vi "UHR-Fleezers Control (host) - 12.2.vi"() -> ()   [LabVIEW 2014] (continued)
          frame #3 {
            n2188 = Wait (ms)(milliseconds to wait=u32 500) -> ()  [unwired: 1 out]
          }
          frame #4 {
            n2189 = property on="Trap Pos. FB ON" class="Bool (strict)"("Val(Sgnl)"=TRUE ("Value (Signaling)")) -> ()  [unwired: 2 in, 2 out]
            n2190 = Wait (ms)(milliseconds to wait=u32 250) -> ()  [unwired: 1 out]
          }
          frame #5 {
            n2191 = case shown="\"1\"" "Remove Action Offset Dropdown" {
              tunnel: TRUE ("Value (Signaling)") -> [w3127 w3135 w3143]
              frame "1" {
                n2192 = flat-sequence {
                  tunnel: w3127 -> [w3134]
                  frame #0 {
                    n2193 = local read "factor"() -> (w3129:dbl)
                    n2194 = Greater Than 0?(x=w3129) -> (x > 0?=w3133:bool)
                    n2195 = Select(t=1.0, s=w3133, f=-1.0) -> (s? t:f=w3130:dbl)
                    n2196 = Multiply(x=w3130, y=w3129) -> (x*y=w3128:dbl)
                    n2197 = local write "factor"(w3128) -> ()
                  }
                  frame #1 {
                    n2198 = property on="Remove Offset to factor" class="Bool (strict)"("Val(Sgnl)"=w3134) -> ()  [unwired: 2 in, 2 out]
                  }
                }
              }
              frame "2" {
                n2199 = flat-sequence {
                  tunnel: w3135 -> [w3142]
                  frame #0 {
                    n2200 = local read "factor"() -> (w3136:dbl)
                    n2201 = Greater Than 0?(x=w3136) -> (x > 0?=w3141:bool)
                    n2202 = Select(t=-1.0, s=w3141, f=1.0) -> (s? t:f=w3139:dbl)
                    n2203 = Multiply(x=w3136, y=w3139) -> (x*y=w3138:dbl)
                    n2204 = local write "factor"(w3138) -> ()
                  }
                  frame #1 {
                    n2205 = property on="Remove Offset to factor" class="Bool (strict)"("Val(Sgnl)"=w3142) -> ()  [unwired: 2 in, 2 out]
                  }
                }
              }
              frame "0", Default {
                n2206 = property on="Remove Action Offset" class="Bool (strict)"("Val(Sgnl)"=w3143) -> ()  [unwired: 2 in, 2 out]
              }
            }
            n2207 = case shown="False" "Trap Trig Fl." {
              frame False {
                n2208 = case shown="True" "Green ON after FB ON?" {
                  selector: "Green ON after FB ON?" -> [_ w3145]
                  frame False {
                  }
                  frame True {
                    n2209 = property on="Green ON/Interlacing" class="Bool (strict)"("Val(Sgnl)"=w3145) -> ()  [unwired: 2 in, 2 out]
                  }
                }
              }
              frame True {
              }
            }
            n2210 = Wait (ms)(milliseconds to wait=u32 250) -> ()  [unwired: 1 out]
          }
          frame #6 {
            n2211 = property on="Start Saving" class="Bool (strict)"("Val(Sgnl)"=TRUE ("Value (Signaling)")) -> ()  [unwired: 2 in, 2 out]
            n2212 = Wait (ms)(milliseconds to wait=u32 5000) -> ()  [unwired: 1 out]
          }
          frame #7 {
            w3149 = TRUE ("Value (Signaling)")
            n2213 = property on="Rem fb disp offset" class="Bool (strict)"("Val(Sgnl)"=w3149) -> ()  [unwired: 2 in, 2 out]
            n2214 = property on="Remove Offset" class="Bool (strict)"("Val(Sgnl)"=w3149) -> ()  [unwired: 2 in, 2 out]
            n2215 = Wait (ms)(milliseconds to wait=u32 100) -> ()  [unwired: 1 out]
          }
          frame #8 {
            n2216 = case shown="True" w3152 {
              frame False {
              }
              frame True {
                n2217 = local write "Trap Trig. Fl."(TRUE ("Value (Signaling)")) -> ()
              }
            }
          }
          frame #9 {
            n2218 = local read "Tether"() -> (w3155:bool)
            n2219 = And(x="Start dipping after?", y=w3155) -> (x .and. y?=w3154:bool)
            n2220 = case shown="True" w3154 {
              frame False {
              }
              frame True {
                n2221 = flat-sequence {
                  frame #0 {
                    n2222 = Multiply(x="Delay before dipping (s)", y=1000.0) -> (x*y=w3158:dbl)
                    n2223 = Wait (ms)(milliseconds to wait=w3158) -> ()  [unwired: 1 out]
                  }
                  frame #1 {
                    n2224 = property on="Dip for Protein" class="Bool (strict)"("Val(Sgnl)"=TRUE ("Value (Signaling)")) -> ()  [unwired: 2 in, 2 out]
                    n2225 = local write "Scripts"(T35."Dipping") -> ()
                  }
                }
              }
            }
          }
        }
      }
      event "Rupture Script": Value Change {
        n2226 = event-data() -> ()  [unwired: 1 in, 5 out]
        n2227 = local write "Rupture Script"(FALSE ("Rupture Script")) -> ()
        n2228 = flat-sequence {
          frame #0 {
            w3164 = TRUE
            w3169 = FALSE
            # "Number 6 for now is the\nrupture-experiment\nparameters."
            n2229 = local read "Starting Trap D (MHz)"() -> (w3170:dbl)
            n2230 = local write "Restart DMA? (AOD)"(w3169) -> ()
            n2231 = Replace Array Subset(array=u32[] [0] ("Index Values"), new element=6, index=0) -> (w3165:u32[])
            n2232 = local write "Save scans"(w3169) -> ()
            n2233 = property on="Trap D (MHz)" class="DigNum (strict)"("Val(Sgnl)"=w3170) -> ()  [unwired: 2 in, 2 out]
            n2234 = property on="Saved AOD Raster Scan Parameter Sets" class="Arr (strict)"("Index Values"=w3165) -> ()  [unwired: 2 in, 2 out]
            n2235 = property on="Start Saving" class="Bool (strict)"("Val(Sgnl)"=w3164) -> ()  [unwired: 2 in, 2 out]
            n2236 = property on="Green ON/Interlacing" class="Bool (strict)"("Val(Sgnl)"=w3164) -> ()  [unwired: 2 in, 2 out]
          }
          frame #1 {
            n2237 = property on="Load parameters" class="Bool (strict)"("Val(Sgnl)"=TRUE ("Value (Signaling)")) -> ()  [unwired: 2 in, 2 out]
          }
        }
      }
      event "Fixed Traps Script": Value Change {
        n2238 = event-data() -> ()  [unwired: 1 in, 5 out]
        n2239 = local write "Fixed Traps Script"(FALSE ("Fixed Traps Data\nScript")) -> ()
        n2240 = flat-sequence {
          frame #0 {
            n2241 = case shown="True" "Green ON" {
              frame False {
              }
              frame True {
                n2242 = property on="Green ON/Interlacing" class="Bool (strict)"("Val(Sgnl)"=TRUE) -> ()  [unwired: 2 in, 2 out]
              }
            }
            n2243 = local write "Offset (nm)"(0.0 ("Offset (nm)")) -> ()
            n2244 = property on="Sample Channel\nFlow" class="Bool (strict)"("Val(Sgnl)"=FALSE ("Value (Signaling)")) -> ()  [unwired: 2 in, 2 out]
            n2245 = property on="Trap D (MHz)" class="DigNum (strict)"("Val(Sgnl)"="Fixed Traps Trap Delta (MHz)") -> ()  [unwired: 2 in, 2 out]
          }
          frame #1 {
            n2246 = Wait (ms)(milliseconds to wait=u32 1000) -> ()  [unwired: 1 out]
          }
          frame #2 {
            n2247 = local write "Start Saving"(TRUE ("Start Saving")) -> ()
          }
          frame #3 {
            n2248 = local read "Bead Sep. Int. Time (s)"() -> (w3180:dbl)
            n2249 = Multiply(x=w3180, y=1000.0) -> (x*y=w3182:dbl)
            n2250 = Wait (ms)(milliseconds to wait=w3182) -> ()  [unwired: 1 out]
          }
          frame #4 {
            n2251 = property on="Remove Offset" class="Bool (strict)"("Val(Sgnl)"=TRUE ("Value (Signaling)")) -> ()  [unwired: 2 in, 2 out]
          }
          frame #5 {
            n2252 = property on="Dip for Protein" class="Bool (strict)"("Val(Sgnl)"="Start dipping after?") -> ()  [unwired: 2 in, 2 out]
          }
        }
      }
      event "Got DNA bead": Value Change {
        n2253 = event-data() -> ()  [unwired: 1 in, 5 out]
        n2254 = flat-sequence {
          frame #0 {
            w3186 = FALSE ("Key Focus")
            n2255 = local read "Daq spot flow on"() -> (w3187:bool)
            n2256 = case shown="True" w3187 {
              frame False {
              }
              frame True {
                n2257 = property on="Sample Channel\nFlow" class="Bool (strict)"("Val(Sgnl)"=TRUE ("Value (Signaling)")) -> ()  [unwired: 2 in, 2 out]
              }
            }
            n2258 = local write "Got DNA bead"(w3186) -> ()
            n2259 = property on="Got DNA bead" class="Bool (strict)"("Key Focus"=w3186) -> ()  [unwired: 2 in, 2 out]
          }
          frame #1 {
            n2260 = property on="Inject Pump 1" class="Bool (strict)"("Val(Sgnl)"=FALSE ("Value (Signaling)")) -> ()  [unwired: 2 in, 2 out]
          }
          frame #2 {
            n2261 = property on="Cal/Data Acq. Spot" class="Bool (strict)"("Val(Sgnl)"=TRUE ("Value (Signaling)")) -> ()  [unwired: 2 in, 2 out]
          }
        }
      }
      event "Take Stepping Data": Value Change {
        n2262 = event-data() -> ()  [unwired: 1 in, 5 out]
        n2263 = local read "Save ave N"() -> (w3199:dbl)
        n2264 = flat-sequence {
          tunnel: w3199 -> [w3201]
          tunnel: [w3201] -> w3194
          tunnel: [w3203] -> w3195
          tunnel: w3194 -> [w3203]
          tunnel: [w3205] -> w3196
          tunnel: w3195 -> [w3205]
          tunnel: [w3208] -> w3197
          tunnel: w3196 -> [w3208]
          tunnel: [w3210] -> w3198
          tunnel: w3197 -> [w3210]
          tunnel: [w3212] -> w3192
          tunnel: w3198 -> [w3212]
          tunnel: w3192 -> [w3215]
          tunnel: [w3215] -> w3191
          tunnel: w3191 -> [w3216]
          tunnel: [w3216] -> w3193
          tunnel: w3193 -> [w3222]
          frame #0 {
            n2265 = property on="Save ave N" class="DigNum (strict)"("Val(Sgnl)"="Save ave factor") -> ()  [unwired: 2 in, 2 out]
          }
          frame #1 {
            n2266 = Wait (ms)(milliseconds to wait=u32 100) -> ()  [unwired: 1 out]
          }
          frame #2 {
            n2267 = local read "Offset 2 Start (MHz)"() -> (w3207:dbl)
            n2268 = property on="Saved AOD Raster Scan Parameter Sets" class="Arr (strict)"("Index Values"=u32[] [2]) -> ()  [unwired: 2 in, 2 out]
            n2269 = property on="Trap D (MHz)" class="DigNum (strict)"("Val(Sgnl)"=w3207) -> ()  [unwired: 2 in, 2 out]
          }
          frame #3 {
            n2270 = property on="Load parameters" class="Bool (strict)"("Val(Sgnl)"=TRUE ("Value (Signaling)")) -> ()  [unwired: 2 in, 2 out]
          }
          frame #4 {
            n2271 = Wait (ms)(milliseconds to wait=u32 100) -> ()  [unwired: 1 out]
          }
          frame #5 {
            n2272 = property on="Trap Raster Scan" class="Bool (strict)"("Val(Sgnl)"=TRUE ("Value (Signaling)")) -> ()  [unwired: 2 in, 2 out]
          }
          frame #6 {
            n2273 = Wait (ms)(milliseconds to wait=u32 1000) -> ()  [unwired: 1 out]
          }
          frame #7 {
            n2274 = while {
              stop <- w3219 stop-if-true
              n2275 = local read "Raster Scanning..."() -> (w3221:bool)
              n2276 = local read "Saving..."() -> (w3220:bool)
              n2277 = Not(x=w3220) -> (.not. x?=w3217:bool)
              n2278 = Not(x=w3221) -> (.not. x?=w3218:bool)
              n2279 = And(x=w3218, y=w3217) -> (x .and. y?=w3219:bool)
            }
          }
          frame #8 {
            n2280 = property on="Save ave N" class="DigNum (strict)"("Val(Sgnl)"=w3222) -> ()  [unwired: 2 in, 2 out]
          }
        }
      }
      event "Step Size (nm)": Value Change {
        n2281 = event-data() -> ()  [unwired: 1 in, 5 out]
        n2282 = flat-sequence {
          frame #0 {
            n2283 = property on="Saved AOD Raster Scan Parameter Sets" class="Arr (strict)"("Index Values"=u32[] [1]) -> ()  [unwired: 2 in, 2 out]
          }
          frame #1 {
            n2284 = Multiply(x="N Steps", y="Step Size (nm)") -> (x*y=w3224:dbl)
            n2285 = property on="Scan Speed AOD (nm/s) 2" class="DigNum (strict)"("Value"="Step Size (nm)") -> ()  [unwired: 2 in, 2 out]
            n2286 = property on="Step Size AOD (nm) 2" class="DigNum (strict)"("Value"="Step Size (nm)") -> ()  [unwired: 2 in, 2 out]
            n2287 = property on="Scan Range AOD (nm) 2" class="DigNum (strict)"("Value"=w3224) -> ()  [unwired: 2 in, 2 out]
          }
        }
      }
      event "Take Detection Laser\nImage": Value Change {
        n2288 = event-data() -> ()  [unwired: 1 in, 5 out]
        n2289 = flat-sequence {
          tunnel: [w3252] -> w3242
          tunnel: [w3251] -> w3235
          tunnel: [w3250] -> w3227
          tunnel: [w3255] -> w3243
          tunnel: w3242 -> [w3255]
          tunnel: [w3254] -> w3236
          tunnel: w3235 -> [w3254]
          tunnel: [w3253] -> w3228
          tunnel: w3227 -> [w3253]
          tunnel: [w3259] -> w3244
          tunnel: w3243 -> [w3259]
          tunnel: [w3258] -> w3237
          tunnel: w3236 -> [w3258]
          tunnel: [w3257] -> w3229
          tunnel: w3228 -> [w3257]
          tunnel: [w3265] -> w3245
          tunnel: w3244 -> [w3265]
          tunnel: [w3264] -> w3238
          tunnel: w3237 -> [w3264]
          tunnel: [w3263] -> w3230
          tunnel: w3229 -> [w3263]
          tunnel: [w3269] -> w3246
          tunnel: w3245 -> [w3269]
          tunnel: [w3268] -> w3239
          tunnel: w3238 -> [w3268]
          tunnel: [w3267] -> w3231
          tunnel: w3230 -> [w3267]
          tunnel: [w3273] -> w3247
          tunnel: w3246 -> [w3273]
          tunnel: [w3272] -> w3240
          tunnel: w3239 -> [w3272]
          tunnel: [w3271] -> w3232
          tunnel: w3231 -> [w3271]
          tunnel: [w3277] -> w3248
          tunnel: w3247 -> [w3277]
          tunnel: [w3276] -> w3241
          tunnel: w3240 -> [w3276]
          tunnel: [w3275] -> w3233
          tunnel: w3232 -> [w3275]
          tunnel: w3248 -> [w3283]
          tunnel: w3241 -> [w3282]
          tunnel: [w3280] -> w3234
          tunnel: w3233 -> [w3280]
          tunnel: w3234 -> [w3284]
          frame #0 {
            n2290 = local read "Laser interlacing mode (all lasers)"() -> (w3251:enum32{"Laser ON", "Laser OFF", "Interlace"})
            n2291 = local read "Green ON/Interlacing"() -> (w3252:bool)
            n2292 = local read "Green FB On/Off"() -> (w3250:bool)
          }
          frame #1 {
            n2293 = property on="Green FB On/Off" class="Bool (strict)"("Val(Sgnl)"=FALSE ("Value (Signaling)")) -> ()  [unwired: 2 in, 2 out]
          }
          frame #2 {
            n2294 = property on="Green ON/Interlacing" class="Bool (strict)"("Val(Sgnl)"=TRUE ("Value (Signaling)")) -> ()  [unwired: 2 in, 2 out]
            n2295 = property on="Flip Green Filter" class="Bool (strict)"("Val(Sgnl)"=TRUE ("Value (Signaling)")) -> ()  [unwired: 2 in, 2 out]
            n2296 = property on="Laser interlacing mode (all lasers)" class="RadioBtnsControl (strict)"("Val(Sgnl)"=enum32{"Laser ON", "Laser OFF", "Interlace"}."Laser ON" ("Value (Signaling)")) -> ()  [unwired: 2 in, 2 out]
          }
          frame #3 {
            n2297 = Wait (ms)(milliseconds to wait=u32 500) -> ()  [unwired: 1 out]
          }
          frame #4 {
            n2298 = property on="Confocal\nImage" class="Bool (strict)"("Val(Sgnl)"=TRUE ("Value (Signaling)")) -> ()  [unwired: 2 in, 2 out]
          }
          frame #5 {
            n2299 = Wait (ms)(milliseconds to wait=u32 2000) -> ()  [unwired: 1 out]
          }
          frame #6 {
            n2300 = while {
              stop <- w3278 stop-if-true
              n2301 = local read "Saving..."() -> (w3279:bool)
              n2302 = Not(x=w3279) -> (.not. x?=w3278:bool)
            }
          }
          frame #7 {
            n2303 = property on="Flip Green Filter" class="Bool (strict)"("Val(Sgnl)"=TRUE ("Value (Signaling)")) -> ()  [unwired: 2 in, 2 out]
            n2304 = property on="Green ON/Interlacing" class="Bool (strict)"("Val(Sgnl)"=w3283) -> ()  [unwired: 2 in, 2 out]
            n2305 = property on="Laser interlacing mode (all lasers)" class="RadioBtnsControl (strict)"("Val(Sgnl)"=w3282) -> ()  [unwired: 2 in, 2 out]
          }
          frame #8 {
            n2306 = property on="Green FB On/Off" class="Bool (strict)"("Val(Sgnl)"=w3284) -> ()  [unwired: 2 in, 2 out]
          }
        }
      }
      event "Stop All": Value Change {
        n2307 = event-data() -> ()  [unwired: 1 in, 5 out]
        n2308 = local read "Stop All"() -> (w3285:bool)
      }
    }
    n2309 = node-c288() -> ()  [unwired: 1 in, 1 out]
  }
  n2310 = node-c288() -> (w139:T26)  [unwired: 4 out]
  n2311 = timed-loop "Mouse control: trap position (AOM deflection), set confocal spot from image" {
    tunnel: [w3287] -> w224
    tunnel: w51 -> [w3286]
    timing: w139 -> [_]
    timing-out: [_] -> w138
    stop <- w3287 stop-if-true
    n2312 = node-c288() -> ()  [unwired: 2 out]
    n2313 = event shown="[0] \"Pane\": Mouse Down" {
      selector: _ -> [_ _]
      dyn-events: _ -> [_ _]
      timeout: _ -> [_ _]
      tunnel: w3286 -> [w3290 _]
      event Mouse Down {
        n2314 = event-data() -> ("Time"=w3292:u32, "Coords"=w3291:T7, "Button"=w3293:u16)  [unwired: 6 out]
        n2315 = case shown="1" w3293 {
          tunnel: w3292 -> [_ _ w3432]
          tunnel: w3291 -> [_ w3298 w3430]
          tunnel: w3290 -> [_ _ w3428]
          frame 0, Default {
          }
          frame 1 {
            n2316 = property on="APD 2" class="ImageControl"() -> ("Displayed Image Position"=w3312:cluster{"Left":i32, "Top":i32})  [unwired: 2 in, 2 out]
            n2317 = control-ref of="Primary Video Display"() -> (w3305:refnum<vi>)
            n2318 = property on="APD 1" class="ImageControl"() -> ("Displayed Image Position"=w3341:cluster{"Left":i32, "Top":i32})  [unwired: 2 in, 2 out]
            n2319 = property on="Detection Laser X" class="ImageControl"() -> ("Displayed Image Position"=w3338:cluster{"Left":i32, "Top":i32})  [unwired: 2 in, 2 out]
            n2320 = property on="Detection Laser Y" class="ImageControl"() -> ("Displayed Image Position"=w3337:cluster{"Left":i32, "Top":i32})  [unwired: 2 in, 2 out]
            n2321 = property on="APD 2" class="ImageControl"() -> ("Displayed Image Size"=w3311:cluster{"Width":u32, "Height":u32})  [unwired: 2 in, 2 out]
            n2322 = property on="APD 1" class="ImageControl"() -> ("Displayed Image Size"=w3339:cluster{"Width":u32, "Height":u32})  [unwired: 2 in, 2 out]
            n2323 = property on="Detection Laser X" class="ImageControl"() -> ("Displayed Image Size"=w3340:cluster{"Width":u32, "Height":u32})  [unwired: 2 in, 2 out]
            n2324 = property on="Detection Laser Y" class="ImageControl"() -> ("Displayed Image Size"=w3336:cluster{"Width":u32, "Height":u32})  [unwired: 2 in, 2 out]
            n2325 = property class="ImageControl"(reference=w3305) -> ("Displayed Image Position"=w3303:cluster{"Left":i32, "Top":i32})  [unwired: 1 in, 2 out]
            n2326 = property class="ImageControl"(reference=w3305) -> ("Displayed Image Size"=w3304:cluster{"Width":u32, "Height":u32})  [unwired: 1 in, 2 out]
            n2327 = Unbundle By Name(w3311) -> ("Width"=w3308:u32, "Height"=w3307:u32)
            n2328 = Unbundle By Name(w3312) -> ("Left"=w3310:i32, "Top"=w3309:i32)
            n2329 = Unbundle By Name(w3339) -> ("Width"=w3333:u32, "Height"=w3332:u32)
            n2330 = Unbundle By Name(w3340) -> ("Width"=w3329:u32, "Height"=w3328:u32)
            n2331 = Unbundle By Name(w3336) -> ("Width"=w3325:u32, "Height"=w3324:u32)
            n2332 = Unbundle By Name(w3341) -> ("Left"=w3335:i32, "Top"=w3334:i32)
            n2333 = Unbundle By Name(w3338) -> ("Left"=w3331:i32, "Top"=w3330:i32)
            n2334 = Unbundle By Name(w3337) -> ("Left"=w3327:i32, "Top"=w3326:i32)
            n2335 = Bundle("Left"=w3310, "Top"=w3309, "Width"=w3308, "Height"=w3307) -> (w3306:T36)  [unwired: 1 in]
            n2336 = Bundle("Left"=w3335, "Top"=w3334, "Width"=w3333, "Height"=w3332) -> (w3323:T36)  [unwired: 1 in]
            n2337 = Bundle("Left"=w3331, "Top"=w3330, "Width"=w3329, "Height"=w3328) -> (w3322:T36)  [unwired: 1 in]
            n2338 = Bundle("Left"=w3327, "Top"=w3326, "Width"=w3325, "Height"=w3324) -> (w3321:T36)  [unwired: 1 in]
            n2339 = Unbundle By Name(w3304) -> ("Width"=w3300:u32, "Height"=w3299:u32)
            n2340 = Unbundle By Name(w3303) -> ("Left"=w3302:i32, "Top"=w3301:i32)
            n2341 = Build Cluster Array(w3306, w3323, w3322, w3321) -> (w3320:T37)
            n2342 = Bundle("Left"=w3302, "Top"=w3301, "Width"=w3300, "Height"=w3299) -> (w3295:T36)  [unwired: 1 in]
            n2343 = for {
              tunnel: w3298 -> [w3374]
              tunnel: w3320 -> [w3375] mode=indexing
              shift-right: [w3372] -> w3318
              shift-left: TRUE -> [w3373]
              shift-right: [w3371] -> w3316
              shift-left: _ -> [w3367]
              shift-right: [w3370] -> w3315
              shift-left: _ -> [w3366]
              shift-right: [w3369] -> w3314
              shift-left: _ -> [w3365]
              shift-right: [w3368] -> w3313
              shift-left: _ -> [w3364]
              n2344 = case shown="True" w3373 {
                selector: w3373 -> [w3380 _]
                tunnel: w3375 -> [_ w3389]
                tunnel: w3374 -> [_ w3387]
                tunnel: [w3380 w3385] -> w3372
                tunnel: [w3379 w3384] -> w3371
                tunnel: [w3378 w3383] -> w3370
                tunnel: [w3377 w3382] -> w3369
                tunnel: [w3376 w3381] -> w3368
                tunnel: w3367 -> [w3379 _]
                tunnel: w3366 -> [w3378 _]
                tunnel: w3365 -> [w3377 _]
                tunnel: w3364 -> [w3376 _]
                frame False {
                }
                frame True {
                  n2345 = Unbundle(w3389) -> (w3388:T36)
                  n2346 = call "isclickinwindow.vi"("Image Param"=w3388, "Point32"=w3387) -> ("4 Y"=w3381:i32, "3 Height"=w3382:i32, "2 X"=w3383:i32, "1 Width"=w3384:i32, "In image?"=w3386:bool)  [unwired: 1 in]
                  n2347 = Not(x=w3386) -> (.not. x?=w3385:bool)
                }
              }
            }
            n2348 = call "isclickinwindow.vi"("Image Param"=w3295, "Point32"=w3298) -> ("4 Y"=w3296:i32, "2 X"=w3297:i32, "In image?"=w3294:bool)  [unwired: 1 in, 2 out]
            n2349 = case shown="True" w3294 {
              tunnel: w3297 -> [_ w3345]
              tunnel: w3296 -> [_ w3348]
              frame False {
              }
              frame True {
                w3357 = 2
                n2350 = Subtract(x=480, y=w3348) -> (x-y=w3347:i32)
                n2351 = Unbundle("Target size") -> ("Width"=w3358:dbl, "Height"=w3356:dbl)
                n2352 = Subtract(x=w3345, y=2) -> (x-y=w3344:i32)
                n2353 = Divide(x=w3356, y=w3357) -> (x/y=w3354:dbl)
                n2354 = Divide(x=w3358, y=w3357) -> (x/y=w3355:dbl)
                n2355 = Subtract(x=w3344, y=w3355) -> (x-y=w3353:dbl)
                n2356 = Add(x=w3344, y=w3355) -> (x+y=w3351:dbl)
                n2357 = Subtract(x=w3347, y=w3354) -> (x-y=w3352:dbl)
                n2358 = Add(x=w3347, y=w3354) -> (x+y=w3350:dbl)
                n2359 = Bundle(w3344, w3347) -> (w3360:cluster{i32, i32})  [unwired: 1 in]
                n2360 = Bundle(w3353, w3352, w3351, w3350) -> (w3342:cluster{dbl, dbl, dbl, dbl})  [unwired: 1 in]
                n2361 = case shown="True" "Set target" {
                  tunnel: w3360 -> [_ w3363]
                  tunnel: w3342 -> [_ w3361]
                  frame False {
                  }
                  frame True {
                    n2362 = local write "Target coordinates"(w3361) -> ()
                    n2363 = local write "Set target"(FALSE ("Set target")) -> ()
                    "Video coordinates" <- w3363
                  }
                }
              }
            }
            n2364 = Not(x=w3318) -> (.not. x?=w3317:bool)
            n2365 = case shown="True" w3317 {
              tunnel: w3315 -> [_ w3403]
              tunnel: w3313 -> [_ w3402]
              tunnel: w3316 -> [_ w3401]
              tunnel: w3314 -> [_ w3400]
              frame False {
              }
              frame True {
                w3390 = FALSE ("Get Point")
                n2366 = local read "Scan lines (y)"() -> (w3405:u64)
                n2367 = disable-structure shown="Disabled" {
                  frame Disabled {
                  }
                  frame Enabled {
                  }
                }
                n2368 = local read "Actual MCL Inc (V)"() -> (w3399:dbl)
                n2369 = local read "Scan steps (MCL)"() -> (w3404:u64)
                n2370 = Divide "Y Pix/step"(x=w3400, y=w3405) -> (x/y=w3412:dbl)
                n2371 = Divide "Y V/pix"(x=w3399, y=w3412) -> (x/y=w3411:dbl)
                n2372 = Divide "Y half step offset"(x=w3399, y=2.0) -> (x/y=w3413:dbl)
                n2373 = Divide "X pix/step"(x=w3401, y=w3404) -> (x/y=w3410:dbl)
                n2374 = Negate(x=w3413) -> (-x=w3414:dbl)
                n2375 = local read "Initial Y"() -> (w3420:dbl)
                n2376 = Multiply(x=w3402, y=w3411) -> (x*y=w3421:dbl)
                n2377 = Divide "X half step offset"(x=w3399, y=2.0) -> (x/y=w3407:dbl)
                n2378 = Divide "X V/pix"(x=w3399, y=w3410) -> (x/y=w3409:dbl)
                n2379 = Multiply(x=w3399, y=w3404) -> (x*y=w3416:dbl)
                n2380 = Compound Arithmetic op=ADD(w3414, w3421, w3420) -> (w3391:dbl)
                "Pointer Y (V)" <- w3391
                n2381 = Multiply(x=w3409, y=w3403) -> (x*y=w3418:dbl)
                n2382 = Negate(x=w3407) -> (-x=w3406:dbl)
                n2383 = local read "Initial X"() -> (w3419:dbl)
                n2384 = Negate(x=w3418) -> (-x=w3417:dbl)
                n2385 = Compound Arithmetic op=ADD(w3406, w3416, w3419, w3417) -> (w3392:dbl)
                "Pointer X (V)" <- w3392
                n2386 = case shown="True" "Set High F Confocal Spot (X-Y)" {
                  tunnel: w3392 -> [_ w3422]
                  tunnel: w3391 -> [_ w3423]
                  frame False {
                  }
                  frame True {
                    "Confocal Y 2 (V)" <- w3423
                    "Confocal X 2 (V)" <- w3422
                  }
                }
                n2387 = Or(x="Set X Only", y="Set Confocal Spot (X-Y)") -> (x .or. y?=w3395:bool)
                n2388 = Or(x="Set Confocal Spot (X-Y)", y="Set Y Only") -> (x .or. y?=w3394:bool)
                n2389 = case shown="True" w3395 {
                  tunnel: w3392 -> [_ w3424]
                  frame False {
                  }
                  frame True {
                    n2390 = property on="AO2" class="Slide (strict)"("Val(Sgnl)"=w3424) -> ()  [unwired: 2 in, 2 out]
                    "Confocal X 1 (V)" <- w3424
                  }
                }
                n2391 = case shown="True" w3394 {
                  tunnel: w3391 -> [_ w3425]
                  frame False {
                  }
                  frame True {
                    n2392 = property on="AO1" class="Slide (strict)"("Val(Sgnl)"=w3425) -> ()  [unwired: 2 in, 2 out]
                    "Confocal Y 1 (V)" <- w3425
                  }
                }
                n2393 = local write "Set High F Confocal Spot (X-Y)"(w3390) -> ()
                n2394 = local write "Set Confocal Spot (X-Y)"(w3390) -> ()
                n2395 = local write "Set X Only"(w3390) -> ()
                n2396 = local write "Set Y Only"(w3390) -> ()
              }
            }
          }
          frame 3 {
            n2397 = local read "BD 2 Frequency 1 (MHz)"() -> (w3426:dbl)
            n2398 = local read "BD 1 Frequency 1 (MHz)"() -> (w3427:dbl)
            n2399 = local write "Manipulating Trap"(TRUE ("Manipulating Trap")) -> ()
            n2400 = local write "Coords"(T7 {"Horizontal"=0, "Vertical"=0} ("Coords")) -> ()
            n2401 = while {
              tunnel: w3432 -> [w3437]
              tunnel: w3430 -> [w3436]
              tunnel: w3428 -> [w3435]
              tunnel: w3427 -> [w3434]
              tunnel: w3426 -> [w3433]
              stop <- w3438 stop-if-true
              n2402 = event shown="[0] \"Pane\": Mouse Move" {
                selector: _ -> [_ _]
                dyn-events: _ -> [_ _]
                timeout: _ -> [_ _]
                tunnel: ["Force Manip Abort" w3502] -> w3438
                tunnel: w3437 -> [w3445 _]
                tunnel: w3436 -> [w3443 _]
                tunnel: w3435 -> [w3442 _]
                tunnel: w3434 -> [w3441 _]
                tunnel: w3433 -> [w3440 _]
                event Mouse Move {
                  n2403 = event-data() -> ("Time"=w3446:u32, "Coords"=w3447:T7)  [unwired: 3 out]
                  n2404 = Less?(x=w3446, y=w3445) -> (x < y?=w3444:bool)
                  n2405 = case "Makes sure old motion events prior to mouse click aren't used" shown="False" w3444 {
                    tunnel: w3447 -> [w3489 _]
                    tunnel: w3443 -> [w3490 _]
                    tunnel: w3442 -> [w3467 _]
                    tunnel: w3441 -> [w3463 _]
                    tunnel: w3440 -> [w3462 _]
                    frame False {
                      n2406 = Subtract(x=w3489, y=w3490) -> (x-y=w3488:T7)
                      "Coords" <- w3488
                      n2407 = local read "Y RF Frequency Limits (MHz)"() -> (w3448:T17)
                      n2408 = To Double Precision Float(number=w3488) -> (double precision float=w3487:cluster{"Horizontal":dbl, "Vertical":dbl})
                      n2409 = Multiply(x=cluster{"Horizontal":dbl, "Vertical":dbl} {"Horizontal"=-1.0, "Vertical"=1.0}, y="Manipulation Scaling") -> (x*y=w3483:cluster{"Horizontal":dbl, "Vertical":dbl})
                      n2410 = local read "X RF Frequency Limits (MHz)"() -> (w3449:T17)
                      n2411 = Multiply(x=w3487, y=w3483) -> (x*y=w3485:cluster{"Horizontal":dbl, "Vertical":dbl})
                      n2412 = Unbundle By Name(w3485) -> ("Horizontal"=w3480:dbl, "Vertical"=w3484:dbl)
                      n2413 = Unbundle By Name(w3448) -> ("Maximum"=w3451:dbl, "Minimum"=w3450:dbl)
                      n2414 = Boolean To (0,1)(Boolean="Manip. X?") -> (0, 1=w3478:i16)
                      n2415 = Boolean To (0,1)(Boolean="Manip. Y?") -> (0, 1=w3475:i16)
                      n2416 = local read "BD 1 Frequency 2 (MHz)"() -> (w3465:dbl)
                      n2417 = Multiply(x=w3484, y=w3475) -> (x*y=w3477:dbl)
                      n2418 = Multiply(x=w3478, y=w3480) -> (x*y=w3481:dbl)
                      n2419 = local read "BD 2 Frequency 2 (MHz)"() -> (w3464:dbl)
                      n2420 = Unbundle By Name(w3449) -> ("Maximum"=w3453:dbl, "Minimum"=w3452:dbl)
                      n2421 = Add(x=w3462, y=w3477) -> (x+y=w3455:dbl)
                      n2422 = Add(x=w3463, y=w3481) -> (x+y=w3457:dbl)
                      n2423 = In Range and Coerce(upper limit=w3453, x=w3457, lower limit=w3452) -> (coerced(x)=w3456:dbl)  [unwired: 1 out]
                      n2424 = In Range and Coerce(upper limit=w3451, x=w3455, lower limit=w3450) -> (coerced(x)=w3454:dbl)  [unwired: 1 out]
                      n2425 = Subtract(x=w3456, y=w3465) -> (x-y=w3474:dbl)
                      n2426 = Subtract(x=w3454, y=w3464) -> (x-y=w3473:dbl)
                      n2427 = Square(x=w3474) -> (x^2=w3472:dbl)
                      n2428 = Square(x=w3473) -> (x^2=w3471:dbl)
                      n2429 = Add(x=w3472, y=w3471) -> (x+y=w3470:dbl)
                      n2430 = Square Root(x=w3470) -> (sqrt(x)=w3466:dbl)
                      n2431 = In Range and Coerce(upper limit="Limit Max (MHz)", x=w3466, lower limit="Limit Min (MHz)") -> (In Range?=w3459:bool)  [unwired: 1 out]
                      n2432 = Not(x="Limits Enable") -> (.not. x?=w3458:bool)
                      n2433 = Or(x=w3459, y=w3458) -> (x .or. y?=w3460:bool)
                      n2434 = case shown="True" w3460 {
                        tunnel: w3467 -> [_ w3500]
                        tunnel: w3466 -> [_ w3491]
                        tunnel: w3456 -> [_ w3498]
                        tunnel: w3465 -> [_ w3497]
                        tunnel: w3454 -> [_ w3496]
                        tunnel: w3464 -> [_ w3495]
                        tunnel: w3449 -> [_ w3493]
                        tunnel: w3448 -> [_ w3492]
                        frame False {
                        }
                        frame True {
                          n2435 = local read "BD 1 Frequency 3 (MHz)"() -> (w3499:dbl)
                          n2436 = local read "BD 2 Frequency 3 (MHz)"() -> (w3494:dbl)
                          n2437 = local write "Trap D (MHz)"(w3491) -> ()
                          n2438 = call "set RF board frequency - interlace.vi"("Board 2 Frequency Limits"=w3492, "Board 1 Frequency Limits"=w3493, "FPGA VI Reference In"=w3500, "Board 2 Frequency 3 (MHz)"=w3494, "Board 1 Frequency 3 (MHz)"=w3499, "Board 2 Frequency 2 (MHz)"=w3495, "Board 2 Frequency 1 (MHz)"=w3496, "Board 1 Frequency 2 (MHz)"=w3497, "Board 1 Frequency 1  (MHz)"=w3498) -> ()  [unwired: 1 in, 2 out]
                          n2439 = local write "BD 2 Frequency 1 (MHz)"(w3496) -> ()
                          n2440 = local write "BD 1 Frequency 1 (MHz)"(w3498) -> ()
                        }
                      }
                    }
                    frame True {
                    }
                  }
                }
                event Mouse Up {
                  n2441 = event-data() -> ("Button"=w3501:u16)  [unwired: 8 out]
                  n2442 = case shown="3" w3501 {
                    tunnel: [FALSE TRUE] -> w3502
                    frame 0, Default {
                    }
                    frame 3 {
                      n2443 = local read "Trap D (MHz)"() -> (w3504:dbl)
                      n2444 = property on="Initial D (MHz)" class="DigNum (strict)"("Val(Sgnl)"=w3504) -> ()  [unwired: 2 in, 2 out]
                      n2445 = local write "Manipulating Trap"(FALSE ("Manipulating Trap")) -> ()
                    }
                  }
                }
              }
            }
          }
        }
      }
      event Mouse Move {
        n2446 = event-data() -> ()  [unwired: 6 out]
      }
    }
    n2447 = local read "Stop All"() -> (w3287:bool)
    n2448 = node-c288() -> ()  [unwired: 2 out]
  }
  n2449 = node-c288(w136) -> ()  [unwired: 1 out]
  n2450 = node-c288(w138) -> ()  [unwired: 1 out]
  n2451 = node-c288(w125) -> ()  [unwired: 1 out]
  n2452 = flat-sequence "Video" {
    tunnel: [w3515] -> w127
    tunnel: w127 -> [w3556]
    frame #0 {
      n2453 = while {
        stop <- w3508 continue-if-true
        n2454 = call "Close Video Capture.vi"() -> ("error code OUT"=w3510:i32)
        n2455 = Equal?(x=w3510, y=0) -> (x = y?=w3508:bool)
      }
      n2456 = local write "Stop All"(FALSE ("Stop All")) -> ()
    }
    frame #1 {
      n2457 = call "DMR_Init.vi"() -> ()  [unwired: 3 out]
    }
    frame #2 {
      # "Setting the destination format to Mono8 makes sure that the image can be displayed in the intensity plot."
      n2458 = call "DMR_GetDevice.vi"("search string IN"="DE019116701") -> ("device handle OUT"=w3533:i32)  [unwired: 4 in, 2 out]
      n2459 = call "DMR_OpenDevice.vi"("device handle IN"=w3533) -> ("driver handle OUT"=w3516:i32)  [unwired: 4 out]
      n2460 = call "DMR_FindList.vi"("flags IN"=u32 0 ("flags"), "list name IN"="" ("String"), "list type IN"=T38."camera descriptions", "driver handle IN"=w3516) -> ("list handle OUT"=w3519:i32)  [unwired: 2 out]
      n2461 = call "DMR_FindList.vi"("flags IN"=u32 0 ("flags"), "list name IN"="Base", "list type IN"=T38."setting", "driver handle IN"=w3516) -> ("list handle OUT"=w3517:i32)  [unwired: 2 out]
      n2462 = call "OBJ_GetHandle.vi"("object name IN"="VideoStandard", "list handle IN"=w3519) -> ("object handle OUT"=w3513:i32)  [unwired: 3 out]
      n2463 = call "OBJ_GetHandle.vi"("object name IN"="PixelFormat", "list handle IN"=w3517) -> ("object handle OUT"=w3527:i32)  [unwired: 3 out]
      n2464 = call "OBJ_SetS.vi"("value index IN"=0, "value IN"="NTSC M", "object handle IN"=w3513) -> ()  [unwired: 2 out]
      n2465 = call "OBJ_SetS.vi"("value index IN"=0, "value IN"="Mono8" ("value"), "object handle IN"=w3527) -> ()  [unwired: 2 out]
      n2466 = call "OBJ_GetHandle.vi"("object name IN"="VideoChannel", "list handle IN"=w3517) -> ("object handle OUT"=w3523:i32)  [unwired: 3 out]
      n2467 = while {
        tunnel: [w3538] -> w3515
        tunnel: w3516 -> [w3535]
        stop <- w3536 continue-if-true
        n2468 = call "DMR_ImageRequestSingle.vi"("request control IN"=0, "driver handle IN"=w3535) -> ("error code OUT"=w3537:i32, "driver handle OUT"=w3538:i32)  [unwired: 2 out]
        n2469 = Equal To 0?(x=w3537) -> (x = 0?=w3536:bool)
      }
      n2470 = call "OBJ_SetI.vi"("value index IN"=0, "value IN"=3 ("Video channel"), "object handle IN"=w3523) -> ()  [unwired: 2 out]
    }
    frame #3 {
      w3544 = T20 0 items=["Grayscale (U8)", "Grayscale (I16)", "Grayscale (SGL)", "Complex (CSG)", "RGB (U32)", "HSL (U32)", "RGB (U64)"] ("Image Type")
      w3552 = T20 0 items=["Grayscale (U8)", "Grayscale (I16)", "Grayscale (SGL)", "Complex (CSG)", "RGB (U32)", "HSL (U32)", "RGB (U64)"] ("Image Type")
      n2471 = for "Create Greyscale map" {
        N: 256 -> [_]
        tunnel: [w3558] -> w3541 mode=indexing
        workers-P: _ -> [_]
        i -> [w3561]
        n2472 = To Unsigned Byte Integer(number=w3561) -> (unsigned 8bit integer=w3557:u8)
        n2473 = Join Numbers(hi=w3557, lo=w3557) -> ((hi.lo)=w3560:u16)
        n2474 = Join Numbers(hi=w3557, lo=w3557) -> ((hi.lo)=w3559:u16)
        n2475 = Join Numbers(hi=w3560, lo=w3559) -> ((hi.lo)=w3558:u32)
      }
      n2476 = call "IMAQ Create"("Image Name"="Scaled video", "Image Type"=w3544) -> ("New Image"=w3543:T2)  [unwired: 2 in, 2 out]
      n2477 = call "IMAQ Create"("Image Name"="Main video", "Image Type"=w3552) -> ("New Image"=w3553:T2)  [unwired: 2 in, 2 out]
      n2478 = node-c288(0 ("Processor")) -> (w3551:T26)  [unwired: 3 out]
      n2479 = Initialize Array(u32 0 ("Window Number (0...15)"), 480 ("dimension size"), 640 ("dimension size")) -> (w3546:u32[][])
      n2480 = timed-loop {
        tunnel: w3556 -> [w3578]
        tunnel: [w3577] -> w3555
        tunnel: w3553 -> [w3576]
        timing: w3551 -> [_]
        timing-out: [_] -> w3550
        tunnel: w3546 -> [w3565]
        tunnel: w3543 -> [w3563]
        tunnel: w3541 -> [w3562]
        stop <- w3564 stop-if-true
        # "This block performs the \nactual image capture."
        n2481 = node-c288() -> ()  [unwired: 2 out]
        n2482 = local read "Stop All"() -> (w3564:bool)
        n2483 = Reciprocal(x="Video Capture Rate (Hz)") -> (1/x=w3568:dbl)
        n2484 = Multiply(x=w3568, y=1000.0) -> (x*y=w3566:dbl)
        n2485 = call "DMR_ImageRequestWaitFor.vi"("queue number IN"=0, "timeout(ms) IN"=500, "driver handle IN"=w3578) -> ("error code OUT"=w3582:i32, "request number OUT"=w3579:i32, "driver handle OUT"=w3580:i32)
        n2486 = feedback #1(T39 refnum ("Avi Refnum")) -> (w3570:T39)
        n2487 = case shown="True" "New Video File" {
          tunnel: [T39 refnum ("Avi Refnum") w3599] -> w3572
          tunnel: [FALSE TRUE] -> w3573
          tunnel: w3570 -> [_ w3595]
          frame False {
          }
          frame True {
            n2488 = call "Create new save file.vi"("Ext"=".avi" ("string"), "Index In"="Video Index") -> ("Path Out"=w3591:path, "Index Out"=w3592:dbl)  [unwired: 1 in]
            "Path Out" <- w3591
            n2489 = Not Equal?(x=w3595, y=T39 refnum ("Avi Refnum")) -> (x != y?=w3596:bool)
            n2490 = Increment(x=w3592) -> (x+1=w3601:dbl)
            n2491 = case shown="True" w3596 {
              tunnel: w3595 -> [_ w3602]
              frame False {
              }
              frame True {
                n2492 = call "IMAQ AVI Close"("Avi Refnum"=w3602) -> ()  [unwired: 1 in, 10 out]
              }
            }
            n2493 = local write "Video Index"(w3601) -> ()
            n2494 = call "IMAQ AVI Create"("Frames Per Second"=u32 30, "AVI Path"=w3591) -> ("Avi Refnum"=w3599:T39)  [unwired: 5 in, 4 out]
          }
        }
        n2495 = Equal To 0?(x=w3582) -> (x = 0?=w3581:bool)
        n2496 = Select(t=w3572, s=w3573, f=w3570) -> (s? t:f=w3571:T39)
        n2497 = feedback-in #1(w3571) -> ()
        n2498 = case shown="True" w3581 {
          tunnel: w3580 -> [w3603 w3630]
          tunnel: w3579 -> [_ w3629]
          tunnel: [w3603 w3626] -> w3577
          tunnel: w3576 -> [_ w3607]
          tunnel: w3565 -> [_ w3614]
          tunnel: w3571 -> [_ w3612]
          tunnel: w3563 -> [_ w3608]
          tunnel: w3562 -> [_ w3609]
          frame False {
          }
          frame True {
            w3620 = u32 0 ("X-offset IN")
            n2499 = call "DMR_GetImageRequestBufferData.vi"("driver handle IN"=w3630, "request number IN"=w3629) -> ("width OUT"=w3619:i32, "height OUT"=w3618:i32, "driver handle OUT"=w3625:i32, "request number OUT"=w3624:i32, "bytes per pixel OUT"=w3621:i32)  [unwired: 13 out]
            n2500 = call "DMR_GetImageRequestBufferImageData.vi"("driver handle IN"=w3625, "request number IN"=w3624, "bytes per pixel IN"=w3621, "X-offset IN"=w3620, "Y-offset IN"=w3620, "height IN"=w3618, "width IN"=w3619) -> ("driver handle OUT"=w3623:u32, "request number OUT"=w3622:u32, "image OUT"=w3615:u32[][])  [unwired: 10 out]
            n2501 = call "DMR_ImageRequestUnlock.vi"("request number IN"=w3622, "driver handle IN"=w3623) -> ("driver handle OUT"=w3628:i32)  [unwired: 1 in, 2 out]
            n2502 = case shown="True" "Averaging" {
              tunnel: w3615 -> [w3671 w3676]
              tunnel: [w3671 w3675] -> w3611
              tunnel: w3614 -> [_ w3673]
              frame False {
              }
              frame True {
                (unwired) 1
                w3681 = 1
                n2503 = feedback #2(w3673) -> (w3672:u32[][])
                n2504 = Add(x=w3676, y=w3672) -> (x+y=w3677:u32[][])
                n2505 = Select(t=w3673, s="Reset Averaging", f=w3677) -> (s? t:f=w3679:u32[][])
                n2506 = feedback-in #2(w3679) -> ()
                n2507 = feedback #3(w3681) -> (w3674:i32)
                n2508 = Divide(x=w3677, y=w3674) -> (x/y=w3678:dbl[][])
                n2509 = Increment(x=w3674) -> (x+1=w3682:i32)
                n2510 = To Unsigned Long Integer(number=w3678) -> (unsigned 32bit integer=w3675:u32[][])
                n2511 = Select(t=w3681, s="Reset Averaging", f=w3682) -> (s? t:f=w3680:i32)
                n2512 = feedback-in #3(w3680) -> ()
              }
            }
            n2513 = call "DMR_ImageRequestSingle.vi"("request control IN"=0, "driver handle IN"=w3628) -> ("driver handle OUT"=w3626:i32)  [unwired: 3 out]
            n2514 = disable-structure shown="Disabled" {
              disable-tunnel: w3611 -> [w3648 _]
              disable-tunnel: w3608 -> [w3647 _]
              frame Disabled {
                n2515 = To Double Precision Float(number=w3648) -> (double precision float=w3646:dbl[][])
                n2516 = In Range and Coerce(upper limit="Intensity Upper", x=w3646, lower limit="Intensity Lower") -> (coerced(x)=w3645:dbl[][])  [unwired: 1 out]
                n2517 = Subtract(x="Intensity Upper", y="Intensity Lower") -> (x-y=w3642:dbl)
                n2518 = Subtract(x=w3645, y="Intensity Lower") -> (x-y=w3643:dbl[][])
                n2519 = Divide(x=w3643, y=w3642) -> (x/y=w3644:dbl[][])
                n2520 = Multiply(x=255.0, y=w3644) -> (x*y=w3640:dbl[][])
                n2521 = To Unsigned Byte Integer(number=w3640) -> (unsigned 8bit integer=w3649:u8[][])
                n2522 = call "IMAQ ArrayToImage"("Image Pixels (U8)"=w3649, "Image"=w3647) -> ("Image Out"=w3636:T2)  [unwired: 4 in, 5 out]
                n2523 = First Call?() -> (First Call?: T/F=w3637:bool)
                n2524 = case shown="True" w3637 {
                  tunnel: w3636 -> [w3650 w3661]
                  frame False {
                    n2525 = flat-sequence {
                      tunnel: w3650 -> [w3656]
                      frame #0 {
                        w3653 = FALSE ("Get/Set Status? (Set)")
                        w3652 = 0 ("Window Number (0...15)")
                        n2526 = call "IMAQ WindSize"("Get/Set Status? (Set)"=w3653, "Window Number"=w3652) -> ("Width & Height out"=→"Window Size":cluster{"Width":i32, "Height":i32})  [unwired: 4 in, 2 out]
                        n2527 = call "IMAQ WindMove"("Window Number (0...15)"=w3652, "Get/Set Status? (Set)"=w3653) -> ("Coordinates (screen)"=→"Window Position":cluster{"X Position":i32, "Y Position":i32})  [unwired: 3 in, 1 out]
                        n2528 = call "IMAQ WindDraw"("Resize to Image Size? (Y)"=FALSE, "Window Number (0...15)"=w3652, "Image"=w3656) -> ()  [unwired: 7 in, 2 out]
                      }
                      frame #1 {
                        n2529 = call "IMAQ WindZoom 2"("Center Point"="Center Point", "Zoom to Fit? (False)"=FALSE, "Zoom Factor"="Zoom Factor") -> ()  [unwired: 5 in, 4 out]
                      }
                    }
                  }
                  frame True {
                    n2530 = flat-sequence {
                      tunnel: w3661 -> [w3664]
                      tunnel: [w3662] -> w3660
                      tunnel: w3660 -> [w3666]
                      frame #0 {
                        w3663 = TRUE ("Resize to Image Size? (Y)")
                        w3662 = 0 ("Window Number (0...15)")
                        n2531 = call "IMAQ WindNonTearing"("Window Number"=w3662, "NonTearing? (True)"=w3663) -> ()  [unwired: 8 in, 2 out]
                        n2532 = call "IMAQ WindDraw"("Resize to Image Size? (Y)"=w3663, "Window Number (0...15)"=w3662, "Image"=w3664) -> ()  [unwired: 7 in, 2 out]
                      }
                      frame #1 {
                        n2533 = call "IMAQ WindSize"("Scrollbars? (N)"=FALSE, "Width & Height"="Initial Window Size", "Window Number"=w3666) -> ()  [unwired: 3 in, 3 out]
                        n2534 = call "IMAQ WindMove"("Window Number (0...15)"=w3666, "Coordinates (screen)"="Initial Window Position") -> ()  [unwired: 3 in, 2 out]
                      }
                    }
                  }
                }
              }
              frame Enabled {
              }
            }
            n2535 = To Unsigned Byte Integer(number=w3611) -> (unsigned 8bit integer=w3610:u8[][])
            n2536 = call "IMAQ ArrayToImage"("Image Pixels (U8)"=w3610, "Image"=w3607) -> ("Image Out"=w3605:T2)  [unwired: 4 in, 5 out]
            n2537 = case shown="True" "Save Video" {
              tunnel: w3612 -> [_ w3670]
              tunnel: w3605 -> [_ w3669]
              frame False {
              }
              frame True {
                n2538 = call "IMAQ AVI Write Frame"("Image"=w3669, "Avi Refnum"=w3670) -> ()  [unwired: 2 in, 8 out]
              }
            }
            n2539 = case shown="True" "Save Image" {
              tunnel: w3610 -> [_ w3685]
              tunnel: w3609 -> [_ w3684]
              frame False {
              }
              frame True {
                n2540 = call <vilib>:"Flatten Pixmap.vi"("colors"=w3684, "8-bit pixmap"=w3685) -> ("image data"=w3691:T40)  [unwired: 4 in, 5 out]
                n2541 = call "Create new save file.vi"("Insert"="video_frame_" ("string"), "Ext"=".bmp" ("string"), "Index In"="Image Index") -> ("Path Out"=w3687:path, "Index Out"=w3692:dbl)
                n2542 = Increment(x=w3692) -> (x+1=w3686:dbl)
                n2543 = local write "Image Index"(w3686) -> ()
                n2544 = call <vilib>:"Write BMP File.vi"("image data"=w3691, "path to BMP file"=w3687) -> ()  [unwired: 1 in, 9 out]
              }
            }
            n2545 = case shown="True" "Target" {
              tunnel: w3605 -> [w3631 w3635]
              tunnel: [w3631 w3633] -> w3604
              frame False {
              }
              frame True {
                n2546 = local read "Target coordinates"() -> (w3632:cluster{"X1":dbl, "Y1":dbl, "X2":dbl, "Y2":dbl})
                n2547 = call "IMAQ Overlay Oval"("Color"=u32 16711680, "Bounding Rectangle"=w3632, "Image"=w3635) -> ("Image Out"=w3633:T2)  [unwired: 7 in, 1 out]
              }
            }
            "Primary Video Display" <- w3604
          }
        }
        n2548 = node-c288(w3566) -> ()  [unwired: 1 out]
      }
      n2549 = node-c288(w3550) -> ()  [unwired: 1 out]
      n2550 = call "DMR_CloseDevice2.vi"("driver handle IN"=w3555) -> ()  [unwired: 1 in, 4 out]
    }
    frame #4 {
      n2551 = call "DMR_Close.vi"() -> ()  [unwired: 1 out]
    }
  }
  n2552 = local write "Offset (nm)"(0.0 ("Offset (nm)")) -> ()
  n2553 = local write "Bead Mean (nm)"(0.0 ("Bead Mean (nm)")) -> ()
  n2554 = local write "Total Volume\nFlowed P1 (uL)"(w45) -> ()
  n2555 = local write "Total Volume\nFlowed Samp (uL)"(w45) -> ()
  n2556 = local write "Total Volume\nFlowed P3 (uL)"(w45) -> ()
  n2557 = node-c288(i64 1 ("Period"), 1 ("Processor")) -> (w217:T26)  [unwired: 2 out]
  n2558 = timed-loop "Acquire Data" {
    tunnel: w51 -> [w4000]
    tunnel: w98 -> [w3999]
    tunnel: [w4029] -> w309
    tunnel: [w4024] -> w307
    timing: w217 -> [_]
    timing-out: [_] -> w216
    tunnel: w116 -> [w3856]
    stop <- "Stop All" stop-if-true
    w3780 = "Initialize"
    w3846 = "NI_ChannelName" ("name")
    # "I think that the conversion\nfrom 'wiggle amp' to nm\nis 0.277 nm/input. So, 1000\nfor an input is 277 nm."
    n2559 = node-c288() -> ()  [unwired: 2 out]
    n2560 = First Call?() -> (First Call?: T/F=w3815:bool)
    n2561 = Or(x="Reset", y=w3815) -> (x .or. y?=w3816:bool)
    n2562 = local read "Flushing P1"() -> (w3735:bool)
    n2563 = case "Reset data stream" shown="True" w3816 {
      tunnel: w4000 -> [w5065 w5073]
      tunnel: w3999 -> [w5064 w5072]
      tunnel: [w5065 w5067] -> w3728
      tunnel: [w5064 w5066] -> w3995
      frame False {
      }
      frame True {
        w5070 = TRUE ("AI to FIFO")
        n2564 = local write "Overflow (data lost)"(FALSE ("Overflow (data lost)")) -> ()
        n2565 = call "reset FPGA DMA.vi"("error in"=w5072, "FPGA VI Reference In"=w5073) -> ("error out"=w5068:errorcluster, "FPGA VI Reference Out"=w5069:T22)
        n2566 = xnode "Read/Write Control"("FPGA VI Reference In"=w5069, "error in"=w5068, "AI to FIFO"=w5070, "APD to FIFO"=w5070) -> ("FPGA VI Reference Out"=w5067:T22, "error out"=w5066:errorcluster)
      }
    }
    n2567 = case shown="True" w3735 {
      frame False {
      }
      frame True {
        n2568 = local read "Flush rate (uL/m) P1"() -> (w4100:dbl)
        n2569 = local read "HP1 Flush Time (s)"() -> (w4106:dbl)
        n2570 = local read "DMA Update Period (s)"() -> (w4093:dbl)
        n2571 = Divide(x=w4100, y=60.0) -> (x/y=w4092:dbl)
        n2572 = feedback #4(0.0) -> (w4095:dbl)
        n2573 = Divide(x=w4106, y=w4093) -> (x/y=w4098:dbl)
        n2574 = feedback #5(0) -> (w4104:i32)
        n2575 = Increment(x=w4104) -> (x+1=w4097:i32)
        n2576 = Multiply(x=w4093, y=w4092) -> (x*y=w4091:dbl)
        n2577 = Greater?(x=w4097, y=w4098) -> (0:w4103:bool)
        n2578 = Compound Arithmetic op=MULTIPLY(w4093, w4097, w4092) -> (→"P1 Flush Volume (uL)":dbl)
        n2579 = Divide(x=w4097, y=w4098) -> (x/y=→"P1 Flushing Bar":dbl)
        n2580 = Add(x=w4091, y=w4095) -> (x+y=w4094:dbl)
        "Total Volume\nFlowed P1 (uL)" <- w4094
        n2581 = feedback-in #4(w4094) -> ()
        n2582 = case shown="True" w4103 {
          tunnel: w4097 -> [w4107 _]
          tunnel: [w4107 0] -> w4102
          frame False {
          }
          frame True {
            w4108 = FALSE ("Flushing P1")
            n2583 = local write "Inject Pump 1"(w4108) -> ()
            n2584 = local write "Flushing P1"(w4108) -> ()
            n2585 = property on="Clear Volume P1" class="Bool (strict)"("Val(Sgnl)"=TRUE ("Value (Signaling)")) -> ()  [unwired: 2 in, 2 out]
          }
        }
        n2586 = feedback-in #5(w4102) -> ()
      }
    }
    n2587 = Or(x="Start AOD Scan", y="Trap Raster Scan") -> (x .or. y?=w3954:bool)
    n2588 = case "Start AOM raster scan" shown="True" w3954 {
      tunnel: w3728 -> [w4915 w4925]
      tunnel: w3995 -> [w4914 w4924]
      tunnel: [w4915 w4918] -> w3720
      tunnel: [w4914 w4917] -> w3994
      frame False {
      }
      frame True {
        n2589 = case shown="True" "Restart DMA? (AOD)" {
          tunnel: [w4963 w4965] -> w4919
          tunnel: [w4962 w4964] -> w4920
          tunnel: w4925 -> [w4963 w4967]
          tunnel: w4924 -> [w4962 w4966]
          frame False {
          }
          frame True {
            n2590 = local write "Overflow (data lost)"(FALSE ("Overflow (data lost)")) -> ()
            n2591 = call "reset FPGA DMA.vi"("error in"=w4966, "FPGA VI Reference In"=w4967) -> ("error out"=w4964:errorcluster, "FPGA VI Reference Out"=w4965:T22)
          }
        }
        n2592 = local write "Trap Raster Scan"(FALSE ("Trap Raster Scan")) -> ()
        n2593 = case shown="False" "Move MCL Also?" {
          tunnel: w4920 -> [w4929 w4957]
          tunnel: w4919 -> [w4930 w4958]
          tunnel: [w4928 w4961] -> w4918
          tunnel: [w4927 w4960] -> w4917
          frame False {
            w4926 = TRUE ("AI to FIFO")
            n2594 = xnode "Read/Write Control"("FPGA VI Reference In"=w4930, "error in"=w4929, "AI to FIFO"=w4926, "APD to FIFO"=w4926, "Start scan"=w4926) -> ("FPGA VI Reference Out"=w4928:T22, "error out"=w4927:errorcluster)
          }
          frame True {
            w4954 = FALSE ("1D or 2D Scan?")
            w4959 = TRUE ("AI to FIFO")
            # "Count for MCL loop"
            # "N total cycles"
            # "N steps"
            # "V_int"
            n2595 = local read "Scan Range (nm)"() -> (w4936:dbl)
            n2596 = local read "Number of F/B Scans (AOD)"() -> (w4953:u16)
            n2597 = Sign(1:w4936) -> (0:w4935:dbl)
            n2598 = Compound Arithmetic op=MULTIPLY(w4936, "MCL Step Position Ratio", "MCL/AOM Scale Tweak") -> (w4940:dbl)
            n2599 = Negate(x=w4935) -> (-x=w4932:dbl)
            n2600 = Multiply(x=w4932, y="MCL Step Increment (V_int)") -> (x*y=w4934:dbl)
            n2601 = Divide(x=w4940, y="MCL X Cal (nm/V)") -> (x/y=w4946:dbl)
            n2602 = Multiply(x=32767.0 ("y"), y=w4946) -> (x*y=w4952:dbl)
            n2603 = local read "Total Counts (ticks)"() -> (w4937:u32)
            n2604 = local read "Cycles/step (AOD)"() -> (w4948:u64)
            n2605 = local read "Scan steps (AOD)"() -> (w4949:u64)
            n2606 = Divide(x=w4952, y=10.0) -> (x/y=w4945:dbl)
            n2607 = Divide(x=w4945, y="MCL Step Increment (V_int)") -> (x/y=w4943:dbl)
            n2608 = Absolute Value(x=w4943) -> (abs(x)=w4931:dbl)
            n2609 = Compound Arithmetic op=MULTIPLY(w4949, w4948, w4937) -> (w4944:u64)
            n2610 = local write "wait to reset values"(w4959) -> ()
            n2611 = local write "MCL Scanning"(w4959) -> ()
            n2612 = Divide(x=w4944, y=w4931) -> (x/y=w4941:dbl)
            "MCL Count" <- w4941
            n2613 = xnode "Read/Write Control"("FPGA VI Reference In"=w4958, "error in"=w4957, "Scan steps (MCL)"=w4931, "Number of scans (MCL)"=w4953, "Cycles per step (MCL)"=u64 1, "Scan freq.  increment (MCL)"=w4934, "1D or 2D Scan?"=w4954, "MCL Scan Axis"=w4954, "Cont. Scan (MCL)"=w4954, "MCL count"=w4941) -> ("FPGA VI Reference Out"=w4956:T22, "error out"=w4955:errorcluster)